vi "Load-CryptoNight-Step3.vi"(8 "error in":errorcluster, 11 "FileName":string="log_file.8.bin") -> (0 "error out":errorcluster, 3 "output cluster":T1={"a"=[17305248937841088298, 17024460552111218704], "b"=[9581029972675991065, 9654787791092207119], "hp_state_in"=array[2097152 elements], "hp_state_out"=array[2097152 elements], "hp_state_in (u64)"=array[262144 elements], "hp_state_out (u64)"=array[262144 elements]} {"a" format="%.0x"; "b" format="%.0x"; "hp_state_in" format="%.0x"; "hp_state_out" format="%.0x"; "hp_state_in (u64)" format="%.0x"; "hp_state_out (u64)" format="%.0x"})   [LabVIEW 2017]
uses:
  Step-3-Data-Type.ctl
panel:
  out "hp_state_out (u64)":u64[](array[numeric]) format="%.0x"
  out "hp_state_in (u64)":u64[](array[numeric]) format="%.0x"
  out "b":u64[](array[numeric]) format="%.0x"
  out "hp_state_out":u8[](array[numeric]) format="%.0x"
  out "a":u64[](array[numeric]) format="%.0x"
  out "hp_state_in":u8[](array[numeric]) format="%.0x"
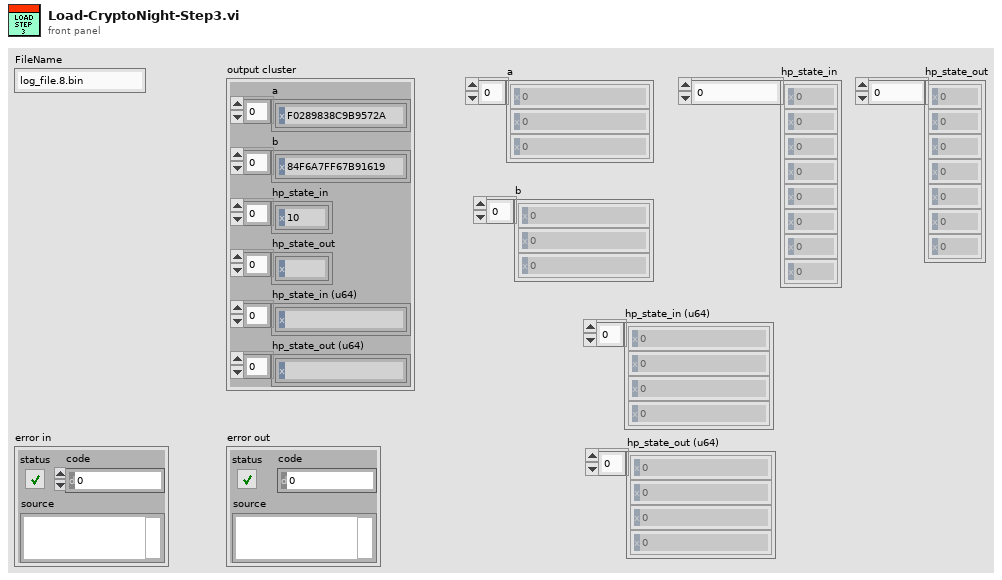
[diagram p1: front panel]
types:
  T1 = typedef "Step-3-Data-Type.ctl" = cluster{"a":u64[], "b":u64[], "hp_state_in":u8[], "hp_state_out":u8[], "hp_state_in (u64)":u64[], "hp_state_out (u64)":u64[]}
  T2 = enum16{"big-endian, network order", "native, host order", "little-endian"}
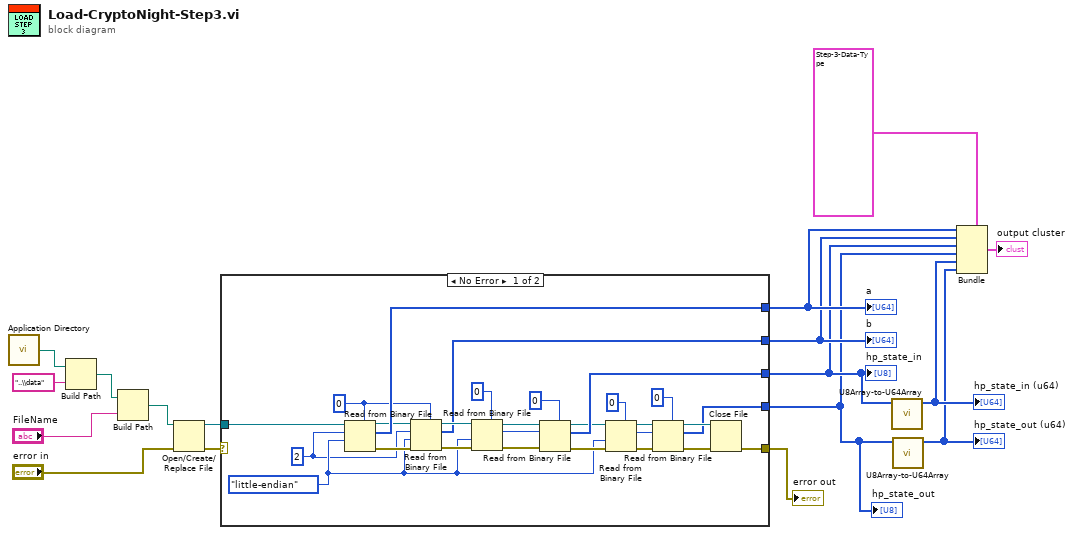
[diagram p0: block diagram]
diagram:
  n1 = call <vilib>:"Application Directory.vi"() -> ("Application Directory"=w9:path)
  n2 = Build Path(base path=w9, name or relative path="..\\data") -> (appended path=w17:path)
  n3 = Build Path(base path=w17, name or relative path="FileName") -> (appended path=w10:path)
  n4 = Open/Create/Replace File(file path (use dialog)=w10, error in="error in") -> (refnum out=w11:refnum<file>, error out=w12:errorcluster)  [unwired: 4 in, 1 out]
  n5 = case shown="No Error" w12 {
    selector: w12 -> [_ w45]
    tunnel: [w41 _] -> w6
    tunnel: [w44 w45] -> w14
    tunnel: [w38 _] -> w8
    tunnel: [w32 _] -> w3
    tunnel: w11 -> [w29 _]
    tunnel: [w18 _] -> w7
    frame No Error {
      w19 = 2 ("count (1)")
      w20 = T2."little-endian" ("byte order (0:big-endian, network order)")
      w23 = u64 0
      n6 = Read from Binary File(5:w23, 9:w20, 10:w19, 11:w29) -> (0:w25:errorcluster, 2:w38:u64[], 3:w22:refnum<file>)  [unwired: 2 in, 1 out]
      n7 = Read from Binary File(5:w23, 8:w25, 9:w20, 10:w19, 11:w22) -> (0:w24:errorcluster, 2:w18:u64[], 3:w21:refnum<file>)  [unwired: 1 in, 1 out]
      n8 = Read from Binary File(5:u32 0, 8:w24, 9:w20, 11:w21) -> (0:w42:errorcluster, 2:w26:u32, 3:w39:refnum<file>)  [unwired: 2 in, 1 out]
      n9 = Read from Binary File(5:u8 0, 8:w42, 10:w26, 11:w39) -> (0:w35:errorcluster, 2:w41:u8[], 3:w30:refnum<file>)  [unwired: 2 in, 1 out]
      n10 = Read from Binary File(5:u32 0, 8:w35, 9:w20, 11:w30) -> (0:w36:errorcluster, 2:w28:u32, 3:w27:refnum<file>)  [unwired: 2 in, 1 out]
      n11 = Read from Binary File(5:u8 0, 8:w36, 10:w28, 11:w27) -> (0:w37:errorcluster, 2:w32:u8[], 3:w34:refnum<file>)  [unwired: 2 in, 1 out]
      n12 = Close File(refnum=w34, error in=w37) -> (error out=w44:errorcluster)  [unwired: 1 out]
    }
    frame Error {
    }
  }
  "hp_state_in" <- w6
  "error out" <- w14
  "a" <- w8
  "hp_state_out" <- w3
  "b" <- w7
  n13 = call "U8Array-to-U64Array.vi"("Array in"=w6) -> ("Array out"=w5:u64[])  [unwired: 10 in]
  "hp_state_in (u64)" <- w5
  n14 = call "U8Array-to-U64Array.vi"("Array in"=w3) -> ("Array out"=w4:u64[])  [unwired: 10 in]
  "hp_state_out (u64)" <- w4
  n15 = Bundle(cluster=T1 {"a"=[17305248937841088298, 17024460552111218704], "b"=[9581029972675991065, 9654787791092207119], "hp_state_in"=array[2097152 elements], "hp_state_out"=array[2097152 elements], "hp_state_in (u64)"=array[262144 elements], "hp_state_out (u64)"=array[262144 elements]} ("CryptoNight-Step-3-Data"), "a"=w8, "b"=w7, "hp_state_in"=w6, "hp_state_out"=w3, "hp_state_in (u64)"=w5, "hp_state_out (u64)"=w4) -> (→"output cluster":T1)
